vi "Simulation Results - Fully Compiled.vi"() -> ()   [LabVIEW 2019]
uses:
  <vilib>/Analysis/NI_AALBase.lvlib
panel:
  out "Numeric":dbl
  out "mean":dbl format="%0.2f"
  out "Color and Time Graph":cluster{dbl[], dbl[]}[](graph)
  out "Full Compiled":T1(array[cluster])
  out "Not Normalized":T2(array[cluster])
  out "Normalized":T2(array[cluster])
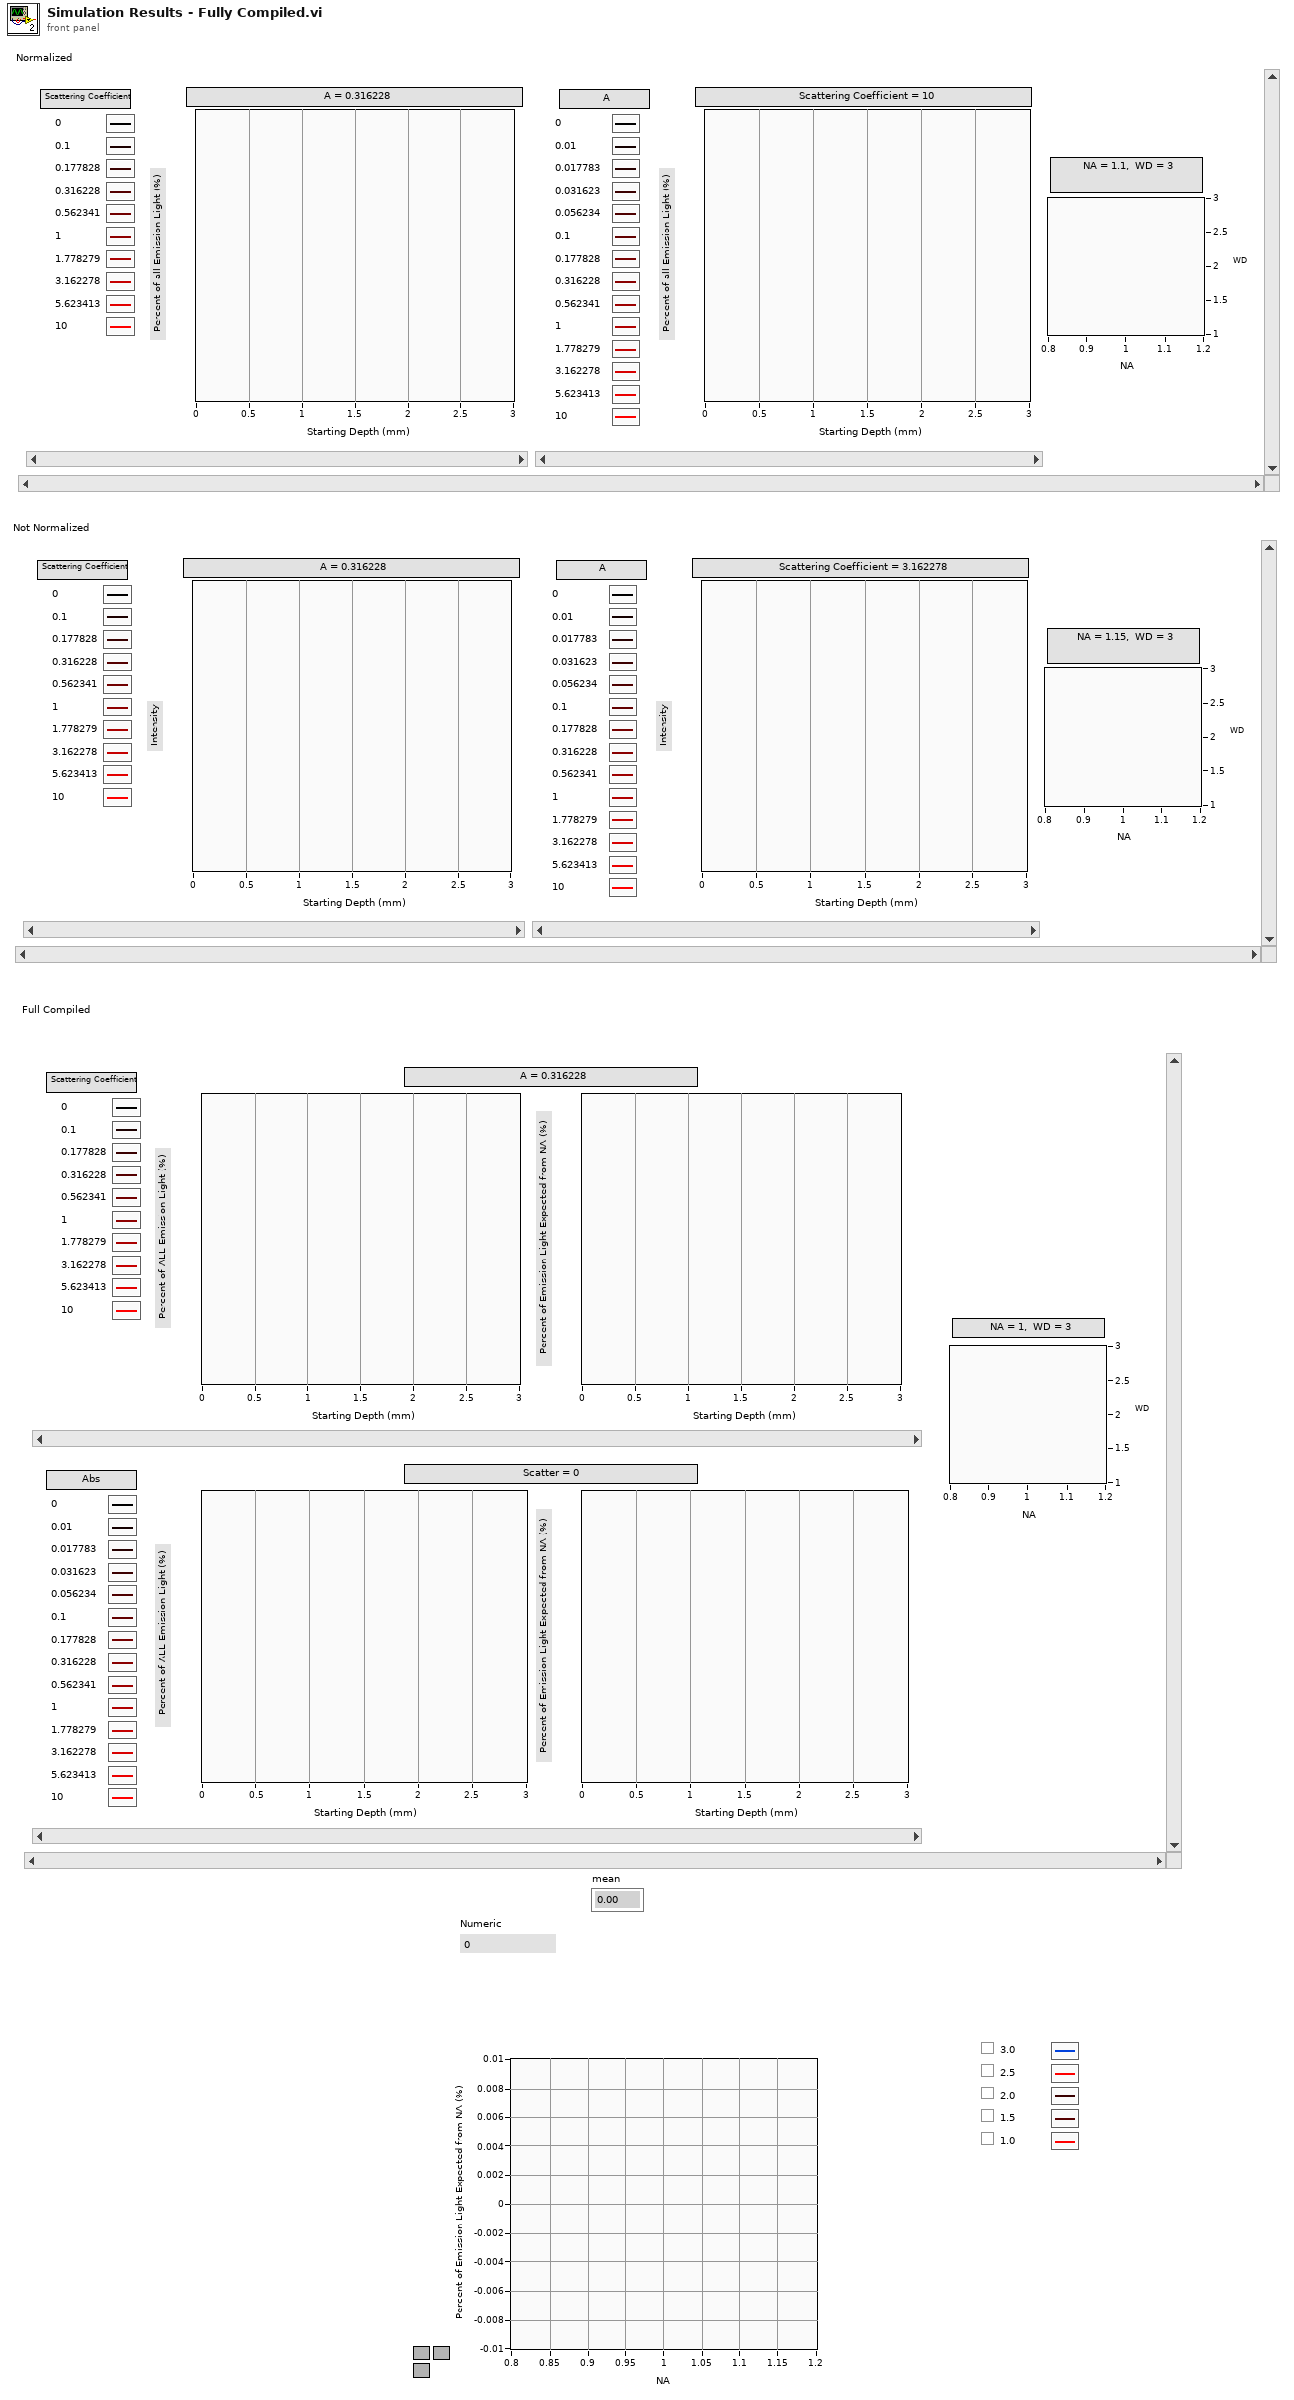
[diagram p1: front panel]
types:
  T1 = cluster{"Slab C=A, T=S 2":cluster{"Color and Time Graph - % RAW":cluster{dbl[], dbl[]}[], "String":string, "String 2":string, "Color and Time Graph":cluster{dbl[], dbl[]}[]}[], "Slab C=A, T=S 2":cluster{"Color and Time Flipped Graph - % RAW":cluster{dbl[], dbl[]}[], "String":string, "String 2":string, "Color and Time Flipped Graph":cluster{dbl[], dbl[]}[]}[], "Supra-Space Label":string, "Supra-Space Mini Map":cluster{dbl[], dbl[]}[]}[][]
  T2 = cluster{"Slab C=A, T=S 2":cluster{"Color and Time Graph":cluster{dbl[], dbl[]}[], "String":string, "String 2":string}[], "Slab C=S, T=A":cluster{"Color and Time Flipped Graph":cluster{dbl[], dbl[]}[], "String":string, "String 2":string}[], "Supra-Space Label":string, "Supra-Space Mini Map":cluster{dbl[], dbl[]}[]}[][]
  T3 = cluster{"Color and Time Graph":cluster{dbl[], dbl[]}[], "String":string, "String 2":string}[]
  T4 = cluster{"Color and Time Flipped Graph":cluster{dbl[], dbl[]}[], "String":string, "String 2":string}[]
  T5 = cluster{"Color and Time Graph":cluster{dbl[], dbl[]}[], "String":string, "String 2":string}
  T6 = cluster{"Color and Time Flipped Graph":cluster{dbl[], dbl[]}[], "String":string, "String 2":string}
  T7 = cluster{"Slab C=A, T=S 2":cluster{"Color and Time Graph":cluster{dbl[], dbl[]}[], "String":string, "String 2":string}[], "Slab C=S, T=A":cluster{"Color and Time Flipped Graph":cluster{dbl[], dbl[]}[], "String":string, "String 2":string}[], "Supra-Space Label":string, "Supra-Space Mini Map":cluster{dbl[], dbl[]}[]}
  T8 = cluster{"Color and Time Graph":cluster{dbl[], dbl[]}[], "String":string, "String 2":string, "Color and Time Graph":cluster{dbl[], dbl[]}[]}
  T9 = cluster{"Color and Time Flipped Graph":cluster{dbl[], dbl[]}[], "String":string, "String 2":string, "Color and Time Flipped Graph":cluster{dbl[], dbl[]}[]}
  T10 = cluster{cluster{"Color and Time Graph":cluster{dbl[], dbl[]}[], "String":string, "String 2":string, "Color and Time Graph":cluster{dbl[], dbl[]}[]}[], cluster{"Color and Time Flipped Graph":cluster{dbl[], dbl[]}[], "String":string, "String 2":string, "Color and Time Flipped Graph":cluster{dbl[], dbl[]}[]}[], "Supra-Space Label":string, "Supra-Space Mini Map":cluster{dbl[], dbl[]}[]}
  T11 = cluster{"Color and Time Graph - % RAW":cluster{dbl[], dbl[]}[], "String":string, "String 2":string, "Color and Time Graph":cluster{dbl[], dbl[]}[]}[]
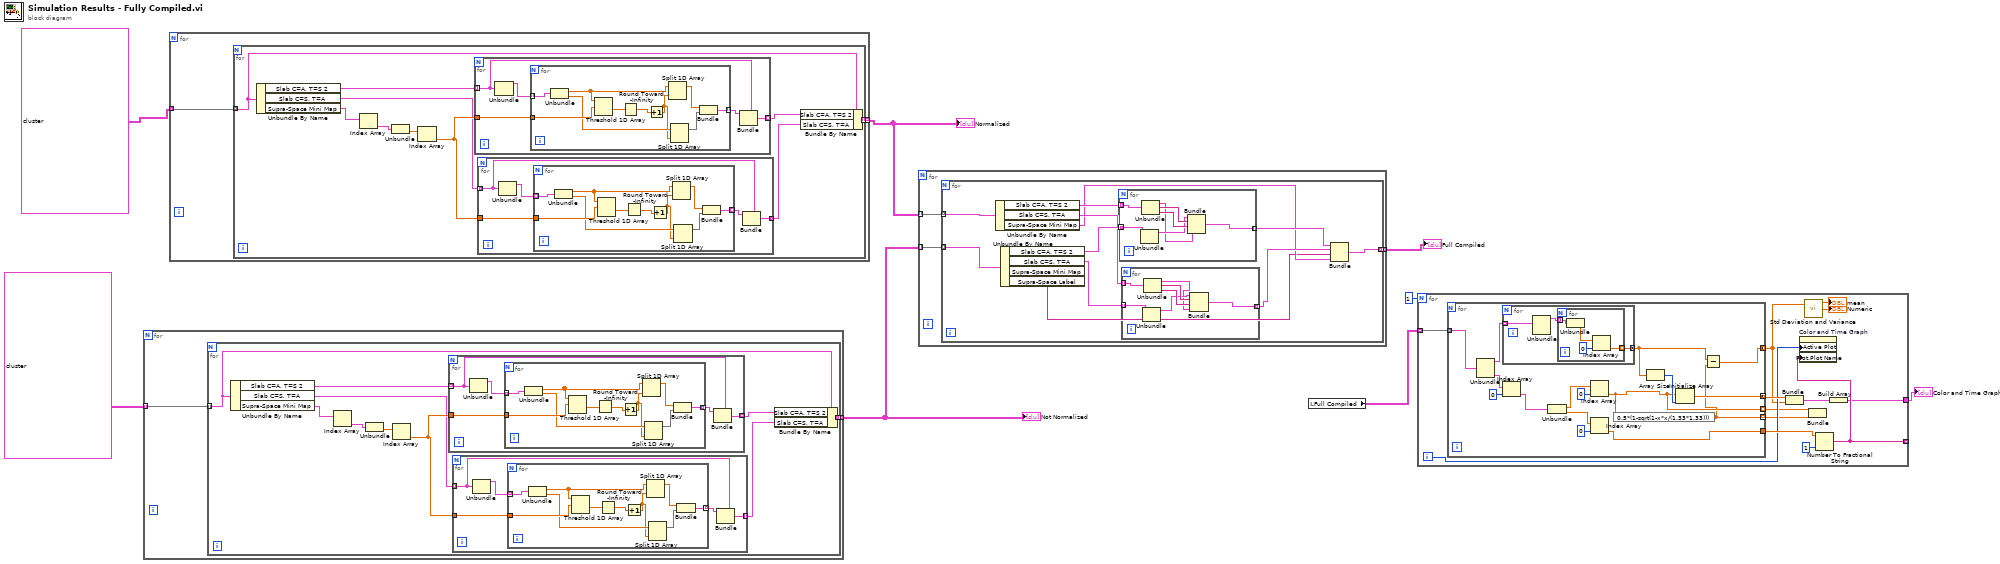
[diagram p0: block diagram]
diagram:
  n1 = for {
    tunnel: T2 data[7241634B] ("Not Normalized") -> [w10] mode=indexing
    tunnel: [w9] -> w5 mode=indexing
    n2 = for {
      tunnel: w10 -> [w16] mode=indexing
      tunnel: [w11] -> w9 mode=indexing
      n3 = Unbundle By Name(w16) -> ("Slab C=A, T=S 2"=w17:T3, "Slab C=S, T=A"=w13:T4, "Supra-Space Mini Map"=w20:cluster{dbl[], dbl[]}[])
      n4 = Index Array(array=w20) -> (element=w19:cluster{dbl[], dbl[]})  [unwired: 1 in]
      n5 = Unbundle(w19) -> (w18:dbl[])  [unwired: 1 out]
      n6 = Index Array(array=w18) -> (element=w14:dbl)  [unwired: 1 in]
      n7 = for {
        tunnel: w17 -> [w38] mode=indexing
        tunnel: w14 -> [w39]
        tunnel: [w36] -> w15 mode=indexing
        n8 = Unbundle(w38) -> ("Color and Time Graph"=w40:cluster{dbl[], dbl[]}[])  [unwired: 2 out]
        n9 = for {
          tunnel: w40 -> [w50] mode=indexing
          tunnel: w39 -> [w49]
          tunnel: [w41] -> w37 mode=indexing
          n10 = Unbundle(w50) -> (w46:dbl[], w45:dbl[])
          n11 = Threshold 1D Array(2:w49, 3:w46) -> (0:w48:dbl)  [unwired: 1 in]
          n12 = Round Toward -Infinity(1:w48) -> (0:w47:dbl)
          n13 = Increment(x=w47) -> (x+1=w44:dbl)
          n14 = Split 1D Array(array=w46, index=w44) -> (first subarray=w43:dbl[])  [unwired: 1 out]
          n15 = Split 1D Array(array=w45, index=w44) -> (first subarray=w42:dbl[])  [unwired: 1 out]
          n16 = Bundle(w43, w42) -> (w41:cluster{dbl[], dbl[]})  [unwired: 1 in]
        }
        n17 = Bundle(cluster=w38, "Color and Time Graph"=w37) -> (w36:T5)  [unwired: 2 in]
      }
      n18 = for {
        tunnel: w13 -> [w23] mode=indexing
        tunnel: w14 -> [w24]
        tunnel: [w21] -> w12 mode=indexing
        n19 = Unbundle(w23) -> ("Color and Time Flipped Graph"=w25:cluster{dbl[], dbl[]}[])  [unwired: 2 out]
        n20 = for {
          tunnel: w25 -> [w35] mode=indexing
          tunnel: w24 -> [w34]
          tunnel: [w26] -> w22 mode=indexing
          n21 = Unbundle(w35) -> (w31:dbl[], w30:dbl[])
          n22 = Threshold 1D Array(2:w34, 3:w31) -> (0:w33:dbl)  [unwired: 1 in]
          n23 = Round Toward -Infinity(1:w33) -> (0:w32:dbl)
          n24 = Increment(x=w32) -> (x+1=w29:dbl)
          n25 = Split 1D Array(array=w31, index=w29) -> (first subarray=w28:dbl[])  [unwired: 1 out]
          n26 = Split 1D Array(array=w30, index=w29) -> (first subarray=w27:dbl[])  [unwired: 1 out]
          n27 = Bundle(w28, w27) -> (w26:cluster{dbl[], dbl[]})  [unwired: 1 in]
        }
        n28 = Bundle(cluster=w23, "Color and Time Flipped Graph"=w22) -> (w21:T6)  [unwired: 2 in]
      }
      n29 = Bundle By Name(cluster=w16, "Slab C=A, T=S 2"=w15, "Slab C=S, T=A"=w12) -> (w11:T7)
    }
  }
  "Not Normalized" <- w5
  n30 = for {
    tunnel: T2 data[7241634B] ("Normalized") -> [w52] mode=indexing
    tunnel: [w51] -> w6 mode=indexing
    n31 = for {
      tunnel: w52 -> [w58] mode=indexing
      tunnel: [w53] -> w51 mode=indexing
      n32 = Unbundle By Name(w58) -> ("Slab C=A, T=S 2"=w59:T3, "Slab C=S, T=A"=w55:T4, "Supra-Space Mini Map"=w62:cluster{dbl[], dbl[]}[])
      n33 = Index Array(array=w62) -> (element=w61:cluster{dbl[], dbl[]})  [unwired: 1 in]
      n34 = Unbundle(w61) -> (w60:dbl[])  [unwired: 1 out]
      n35 = Index Array(array=w60) -> (element=w56:dbl)  [unwired: 1 in]
      n36 = for {
        tunnel: w59 -> [w80] mode=indexing
        tunnel: w56 -> [w81]
        tunnel: [w78] -> w57 mode=indexing
        n37 = Unbundle(w80) -> ("Color and Time Graph"=w82:cluster{dbl[], dbl[]}[])  [unwired: 2 out]
        n38 = for {
          tunnel: w82 -> [w92] mode=indexing
          tunnel: w81 -> [w91]
          tunnel: [w83] -> w79 mode=indexing
          n39 = Unbundle(w92) -> (w88:dbl[], w87:dbl[])
          n40 = Threshold 1D Array(2:w91, 3:w88) -> (0:w90:dbl)  [unwired: 1 in]
          n41 = Round Toward -Infinity(1:w90) -> (0:w89:dbl)
          n42 = Increment(x=w89) -> (x+1=w86:dbl)
          n43 = Split 1D Array(array=w88, index=w86) -> (first subarray=w85:dbl[])  [unwired: 1 out]
          n44 = Split 1D Array(array=w87, index=w86) -> (first subarray=w84:dbl[])  [unwired: 1 out]
          n45 = Bundle(w85, w84) -> (w83:cluster{dbl[], dbl[]})  [unwired: 1 in]
        }
        n46 = Bundle(cluster=w80, "Color and Time Graph"=w79) -> (w78:T5)  [unwired: 2 in]
      }
      n47 = for {
        tunnel: w55 -> [w65] mode=indexing
        tunnel: w56 -> [w66]
        tunnel: [w63] -> w54 mode=indexing
        n48 = Unbundle(w65) -> ("Color and Time Flipped Graph"=w67:cluster{dbl[], dbl[]}[])  [unwired: 2 out]
        n49 = for {
          tunnel: w67 -> [w77] mode=indexing
          tunnel: w66 -> [w76]
          tunnel: [w68] -> w64 mode=indexing
          n50 = Unbundle(w77) -> (w73:dbl[], w72:dbl[])
          n51 = Threshold 1D Array(2:w76, 3:w73) -> (0:w75:dbl)  [unwired: 1 in]
          n52 = Round Toward -Infinity(1:w75) -> (0:w74:dbl)
          n53 = Increment(x=w74) -> (x+1=w71:dbl)
          n54 = Split 1D Array(array=w73, index=w71) -> (first subarray=w70:dbl[])  [unwired: 1 out]
          n55 = Split 1D Array(array=w72, index=w71) -> (first subarray=w69:dbl[])  [unwired: 1 out]
          n56 = Bundle(w70, w69) -> (w68:cluster{dbl[], dbl[]})  [unwired: 1 in]
        }
        n57 = Bundle(cluster=w65, "Color and Time Flipped Graph"=w64) -> (w63:T6)  [unwired: 2 in]
      }
      n58 = Bundle By Name(cluster=w58, "Slab C=A, T=S 2"=w57, "Slab C=S, T=A"=w54) -> (w53:T7)
    }
  }
  "Normalized" <- w6
  n59 = for {
    tunnel: w6 -> [w95] mode=indexing
    tunnel: w5 -> [w94] mode=indexing
    tunnel: [w93] -> w4 mode=indexing
    n60 = for {
      tunnel: w95 -> [w101] mode=indexing
      tunnel: w94 -> [w106] mode=indexing
      tunnel: [w98] -> w93 mode=indexing
      n61 = Unbundle By Name(w101) -> ("Slab C=A, T=S 2"=w102:T3, "Slab C=S, T=A"=w103:T4, "Supra-Space Mini Map"=w97:cluster{dbl[], dbl[]}[])
      n62 = Unbundle By Name(w106) -> ("Slab C=A, T=S 2"=w105:T3, "Slab C=S, T=A"=w104:T4, "Supra-Space Label"=w96:string)  [unwired: 1 out]
      n63 = for {
        tunnel: w102 -> [w119] mode=indexing
        tunnel: w105 -> [w120] mode=indexing
        tunnel: [w116] -> w100 mode=indexing
        n64 = Unbundle(w120) -> ("Color and Time Graph"=w115:cluster{dbl[], dbl[]}[])  [unwired: 2 out]
        n65 = Unbundle(w119) -> ("Color and Time Graph"=w114:cluster{dbl[], dbl[]}[], "String"=w118:string, "String 2"=w117:string)
        n66 = Bundle("Color and Time Graph"=w115, "String"=w118, "String 2"=w117, "Color and Time Graph"=w114) -> (w116:T8)  [unwired: 1 in]
      }
      n67 = for {
        tunnel: w103 -> [w112] mode=indexing
        tunnel: w104 -> [w113] mode=indexing
        tunnel: [w109] -> w99 mode=indexing
        n68 = Unbundle(w113) -> ("Color and Time Flipped Graph"=w108:cluster{dbl[], dbl[]}[])  [unwired: 2 out]
        n69 = Unbundle(w112) -> ("Color and Time Flipped Graph"=w107:cluster{dbl[], dbl[]}[], "String"=w111:string, "String 2"=w110:string)
        n70 = Bundle("Color and Time Flipped Graph"=w108, "String"=w111, "String 2"=w110, "Color and Time Flipped Graph"=w107) -> (w109:T9)  [unwired: 1 in]
      }
      n71 = Bundle(w100, w99, "Supra-Space Label"=w96, "Supra-Space Mini Map"=w97) -> (w98:T10)  [unwired: 1 in]
    }
  }
  "Full Compiled" <- w4
  n72 = local read "Full Compiled"() -> (w3:T1)
  n73 = for {
    N: 1 -> [_]
    tunnel: w3 -> [w133] mode=indexing
    tunnel: [w124] -> w2
    tunnel: [w128] -> _ mode=indexing
    i -> [w127]
    n74 = for {
      tunnel: w133 -> [w149] mode=indexing
      tunnel: [w139] -> w132 mode=concatenating
      tunnel: [w134] -> w123 mode=concatenating
      tunnel: [w138] -> w130
      tunnel: [w135] -> w125 mode=indexing
      tunnel: [w137] -> w126 mode=indexing
      n75 = Unbundle(w149) -> ("Slab C=A, T=S 2"=w146:T11, "Supra-Space Mini Map"=w148:cluster{dbl[], dbl[]}[])  [unwired: 2 out]
      n76 = Index Array(array=w148, index=0) -> (element=w145:cluster{dbl[], dbl[]})
      n77 = for {
        tunnel: w146 -> [w152] mode=indexing
        tunnel: [w150] -> w136 mode=concatenating
        n78 = Unbundle(w152) -> ("Color and Time Graph - % RAW"=w151:cluster{dbl[], dbl[]}[])  [unwired: 3 out]
        n79 = for {
          tunnel: w151 -> [w155] mode=indexing
          tunnel: [w153] -> w150 mode=indexing
          n80 = Unbundle(w155) -> (w154:dbl[])  [unwired: 1 out]
          n81 = Index Array(array=w154, index=0) -> (element=w153:dbl)
        }
      }
      n82 = Unbundle(w145) -> (w141:dbl[], w142:dbl[])
      n83 = Index Array(array=w141, index=0) -> (element=w137:dbl)
      n84 = Index Array(array=w142, index=0) -> (element=w138:dbl)
      n85 = expression code="0.5*(1-sqrt(1-x*x/(1.33*1.33)))"(w137) -> (w135:dbl)
      n86 = Array Size(array=w136) -> (size(s)=w140:i32)
      n87 = Initialize Array(w137, w140) -> (w139:dbl[])
      n88 = Subtract(x=w136, y=w135) -> (x-y=w134:dbl[])
    }
    n89 = Bundle(w132, w123) -> (w131:cluster{dbl[], dbl[]})  [unwired: 1 in]
    n90 = call <vilib>:"Std Deviation and Variance.vi"("X"=w123) -> ("mean"=→"mean":dbl, "standard deviation"=→"Numeric":dbl)  [unwired: 1 in, 1 out]
    n91 = Bundle(w126, w125) -> ()  [unwired: 1 in, 1 out]
    n92 = Number To Fractional String(number=w130, precision (6)=i16 1) -> (F-format string=w128:string)  [unwired: 2 in]
    n93 = property on="Color and Time Graph" class="XYGraph (strict)"("Active Plot"=w127, "Plot.Plot Name"=w128) -> ()  [unwired: 2 in, 2 out]
    n94 = Build Array(w131) -> (w124:cluster{dbl[], dbl[]}[])
  }
  "Color and Time Graph" <- w2
